vi "HFRR ADV v043.vi"() -> ()   [LabVIEW 2025] (continued)
                  n3190 = call-dynamic "Set Report Tab Width.vi"("report in"=w4006, "error in (no error)"=w4004) -> ("report out"=w4005:refnum<class "NI_report.lvclass">, "error out"=w4003:errorcluster)  [unwired: 12 in]
                }
                n3191 = local read "TITTLE"() -> (w3951:string)
                n3192 = call-dynamic "Set Report Header Text.vi"("report in"=w3934, "center header text"=w3951, "error in (no error)"=w3933) -> ("report out"=w3972:refnum<class "NI_report.lvclass">, "error out"=w3971:errorcluster)  [unwired: 11 in]
                n3193 = for {
                  N: 1 -> [_]
                  tunnel: [w4010] -> w3958
                  tunnel: [w4009] -> w3957
                  tunnel: w3972 -> [w4008]
                  tunnel: w3971 -> [w4007]
                  n3194 = call-dynamic "New Report Line.vi"("report in"=w4008, "error in (no error)"=w4007) -> ("report out"=w4010:refnum<class "NI_report.lvclass">, "error out"=w4009:errorcluster)  [unwired: 12 in]
                }
                n3195 = for {
                  N: 2 -> [_]
                  tunnel: [w4002] -> w3964
                  tunnel: [w4001] -> w3963
                  tunnel: w3958 -> [w4000]
                  tunnel: w3957 -> [w3999]
                  n3196 = call-dynamic "New Report Line.vi"("report in"=w4000, "error in (no error)"=w3999) -> ("report out"=w4002:refnum<class "NI_report.lvclass">, "error out"=w4001:errorcluster)  [unwired: 12 in]
                }
                n3197 = for {
                  N: 25 -> [_]
                  tunnel: w3964 -> [w3998]
                  tunnel: w3963 -> [w3996]
                  tunnel: [w3997] -> w3967
                  tunnel: [w3995] -> w3966
                  n3198 = call-dynamic "Set Report Tab Width.vi"("report in"=w3998, "error in (no error)"=w3996) -> ("report out"=w3997:refnum<class "NI_report.lvclass">, "error out"=w3995:errorcluster)  [unwired: 12 in]
                }
                n3199 = control-ref of="Tab Control 9"() -> (w3962:refnum<vi>)
                n3200 = call-dynamic "Append Control Image to Report.vi"("report in"=w3967, "alignment (default)"=HTML_Report_Image_Alignment."ABSMIDDLE", "ctrl reference"=w3962, "error in (no error)"=w3966) -> ("report out"=w3961:refnum<class "NI_report.lvclass">, "error out"=w3960:errorcluster)  [unwired: 8 in, 2 out]
                n3201 = for {
                  N: 3 -> [_]
                  tunnel: [w3994] -> w3945
                  tunnel: [w3993] -> w3944
                  tunnel: w3961 -> [w3992]
                  tunnel: w3960 -> [w3991]
                  n3202 = call-dynamic "New Report Line.vi"("report in"=w3992, "error in (no error)"=w3991) -> ("report out"=w3994:refnum<class "NI_report.lvclass">, "error out"=w3993:errorcluster)  [unwired: 12 in]
                }
                n3203 = for {
                  N: 100 -> [_]
                  tunnel: w3945 -> [w3990]
                  tunnel: w3944 -> [w3988]
                  tunnel: [w3989] -> w3941
                  tunnel: [w3987] -> w3939
                  n3204 = call-dynamic "Set Report Tab Width.vi"("report in"=w3990, "error in (no error)"=w3988) -> ("report out"=w3989:refnum<class "NI_report.lvclass">, "error out"=w3987:errorcluster)  [unwired: 12 in]
                }
                n3205 = String To Path(string="C:\\LAB-IQ\\im\\Temp_resized.jpg") -> (path=w3931:path)
                n3206 = call-poly <vilib>:"Append Image to Report.vi"("report in"=w3941, "path or URL of image"=w3931, "error in (no error)"=w3939) -> ("report out"=w3940:refnum<class "NI_report.lvclass">, "error out"=w3938:errorcluster)  [unwired: 9 in, 2 out]
                n3207 = call-poly <vilib>:"Open HTML Report in Browser.vi"("report in"=w3940, "error in (no error)"=w3938) -> ("report out"=w3975:refnum<class "NI_report.lvclass">, "error out"=w3974:errorcluster)  [unwired: 11 in, 1 out]
                n3208 = call-dynamic "Dispose Report.vi"("report in"=w3975, "error in (no error)"=w3974) -> ()  [unwired: 13 in, 1 out]
              }
              frame #2 {
              }
              frame #3 {
                n3209 = disable-structure shown="Disabled" {
                  frame Disabled {
                    n3210 = local read "String 10"() -> (w4015:string)
                    n3211 = Concatenate Strings("C:\\LAB-IQ-NXT\\Data\\" ("string"), w4015, ".jpg" ("string")) -> (w4013:string)
                    n3212 = String To Path(string=w4013) -> (path=w4012:path)
                    n3213 = Delete(path (use dialog)=w4012) -> ()  [unwired: 4 in, 3 out]
                  }
                  frame Enabled {
                  }
                }
                n3214 = local write "Print 2"(FALSE ("Print")) -> ()
              }
            }
          }
        }
      }
    }
    n3215 = Wait (ms)(milliseconds to wait=u32 50) -> ()  [unwired: 1 out]
    n3216 = Wait (ms)(milliseconds to wait=u32 50) -> ()  [unwired: 1 out]
    n3217 = local read "Quit"() -> (w2357:bool)
  }
  n3218 = VISA Close(VISA resource name=w45, error in (no error)=w44) -> ()  [unwired: 1 out]
  n3219 = while {
    stop <- w4166 stop-if-true
    n3220 = local read "Auto Start Test"() -> (w4164:bool)
    n3221 = local read "RUN"() -> (w4163:bool)
    n3222 = Wait (ms)(milliseconds to wait=u32 1000) -> ()  [unwired: 1 out]
    n3223 = Or(x=w4163, y=w4164) -> (x .or. y?=w4162:bool)
    n3224 = case shown="True" w4162 {
      frame False {
      }
      frame True {
        n3225 = local read "LVDT STROKE Actual"() -> (w4167:dbl)
        n3226 = In Range and Coerce(upper limit=1.2, x=w4167, lower limit=0.6) -> (In Range?=w4170:bool)  [unwired: 1 out]
        n3227 = call-poly <vilib>:"Random Number (Range).vi"("lower bound (0)"=0.998 ("upper bound (100)"), "upper bound (100)"=1.003) -> ("number"=w4168:dbl)  [unwired: 9 in]
        n3228 = case shown="True" w4170 {
          tunnel: [w4175 w4176] -> w4169
          tunnel: w4168 -> [_ w4176]
          tunnel: w4167 -> [w4175 _]
          frame False {
          }
          frame True {
          }
        }
        "LVDT STROKE DISPLAY" <- w4169
      }
    }
    n3229 = local read "Quit"() -> (w4166:bool)
  }
  n3230 = while {
    tunnel: [w4193] -> w53
    shift-right: [w4186] -> _
    shift-left: 0.0 -> [w4189]
    shift-right: [w4185] -> _
    shift-left: 0.0 -> [w4188]
    shift-right: [w4184] -> _
    shift-left: 100.0 ("vc_cmd") -> [w4187]
    stop <- w4193 stop-if-true
    # "PID LOGIC"
    n3231 = local read "run test Calibration"() -> (w4181:bool)
    n3232 = local read "RUN"() -> (w4191:bool)
    n3233 = local read "Auto Start Temp"() -> (w4182:bool)
    n3234 = local read "Auto Start Test"() -> (w4190:bool)
    n3235 = local read "START TEMP"() -> (w4180:bool)
    n3236 = And(x=w4182, y=w4190) -> (x .and. y?=w4183:bool)
    n3237 = Or(x=w4191, y=w4183) -> (x .or. y?=w4192:bool)
    n3238 = And(x=w4192, y=w4180) -> (x .and. y?=w4179:bool)
    n3239 = And(x=w4181, y=w4180) -> (x .and. y?=w4178:bool)
    n3240 = Or(x=w4178, y=w4179) -> (x .or. y?=w4177:bool)
    n3241 = Wait (ms)(milliseconds to wait="milliseconds to wait") -> ()  [unwired: 1 out]
    n3242 = case shown="True" w4177 {
      tunnel: [400.0 ("out_vc_cmd") w4212] -> w4184
      tunnel: [w4196 w4214] -> w4185
      tunnel: [w4196 w4213] -> w4186
      tunnel: w4189 -> [_ w4203]
      tunnel: w4188 -> [_ w4202]
      tunnel: w4187 -> [_ w4201]
      tunnel: w4181 -> [_ w4197]
      frame False {
        w4196 = 0.0 ("error_out")
      }
      frame True {
        n3243 = case shown="True" w4197 {
          tunnel: [w4221 1.0] -> w4199
          frame False {
            n3244 = local read "Set Strk"() -> (w4220:dbl)
            n3245 = Add(x=w4220, y="Add up Stroke") -> (x+y=w4221:dbl)
          }
          frame True {
          }
        }
        n3246 = local read "LVDT STROKE"() -> (w4198:dbl)
        n3247 = formula code="// Zero-Hardcode Explicit Positional-Form PID Engine\n// Inputs: target_stroke, measured_stroke, dt, prev_error, integral_accumulator_in, prev_vc_cmd\n//         kp, ki, kd, max_step_change, max_amplitude, min_amplitude, startup_cmd\n// Outputs: vc_cmd, error_out, out_error, integral_accumulator_out, out_vc_cmd\n\n// 1. Calculate Tracking Error\nfloat current_error = target_stroke - measured_stroke;\nerror_out = current_error;\n\n// 2. Compute Proportional Term\nfloat p_term = kp * current_error;\n\n// 3. Compute Derivative Term\nfloat d_term = 0.0;\nif (dt > 0.0) {\n    d_term = kd * ((current_error - prev_error) / dt);\n}\n\n// 4. Update and Accumulate Integral Term\nfloat current_integral = integral_accumulator_in + (current_error * dt);\nfloat i_term = ki * current_integral;\n\n// 5. Calculate Ideal Target Command (Anchored by startup baseline)\nfloat ideal_command = startup_cmd + p_term + i_term + d_term;\n\n// 6. Apply Loop Rate Limiting FIRST \n// (Forces the command to climb gradually from prev_vc_cmd instead of jumping straight to max)\nfloat raw_adjustment = ideal_command - prev_vc_cmd;\n\nif (raw_adjustment > max_step_change) {\n    raw_adjustment = max_step_change;\n} else if (raw_adjustment < -max_step_change) {\n    raw_adjustment = -max_step_change;\n}\n\nfloat next_vc_cmd = prev_vc_cmd + raw_adjustment;\n\n// 7. Anti-Windup Protection & Final Output Safety Safeguard Clamping\n// (Back-calculating based on what we are ACTUALLY outputting)\nif (next_vc_cmd > max_amplitude) {\n    float excess = next_vc_cmd - max_amplitude;\n    if (ki > 0.0) {\n        current_integral -= excess / ki;\n    }\n    next_vc_cmd = max_amplitude;\n} else if (next_vc_cmd < min_amplitude) {\n    float excess = next_vc_cmd - min_amplitude;\n    if (ki > 0.0) {\n        current_integral -= excess / ki;\n    }\n    next_vc_cmd = min_amplitude;\n}\n\n// 8. Map to Shift Registers for memory persistence\nvc_cmd = next_vc_cmd;\nout_error = current_error;                   \nintegral_accumulator_out = current_integral;  \nout_vc_cmd = next_vc_cmd;"("target_stroke"=w4199, "measured_stroke"=w4198, "dt"="dt", "integral_accumulator_in"=w4202, "prev_error"=w4203, "prev_vc_cmd"=w4201, "kp"="kp", "ki"="ki", "kd"="kd", "max_step_change"="max_step_change", "max_amplitude"="max_amplitude", "min_amplitude"="min_amplitude", "startup_cmd"="startup_cmd") -> ("vc_cmd"=w4218:dbl, "out_error"=w4213:dbl, "integral_accumulator_out"=w4214:dbl, "out_vc_cmd"=w4212:dbl)  [unwired: 1 out]
        "output Vpp" <- w4218
        n3248 = Number To Fractional String(number=w4218, precision (6)=i16 1) -> (F-format string=w4216:string)  [unwired: 2 in]
        n3249 = Concatenate Strings("DAC;" ("string"), w4216) -> (w4200:string)
        n3250 = local write "Due Write"(w4200) -> ()
        "prev_error" <- w4203
        "integral_accumulator_in" <- w4202
        "prev_vc_cmd" <- w4201
      }
    }
    n3251 = local read "Quit"() -> (w4193:bool)
  }
  n3252 = Or(x=w49, y=w48) -> (x .or. y?=w50:bool)
  n3253 = Or(x=w46, y=w50) -> (x .or. y?=w55:bool)
  n3254 = control-ref of="new picture"() -> ()  [unwired: 1 out]
  n3255 = Or(x=w58, y=w55) -> (x .or. y?=w52:bool)
  n3256 = Or(x=w52, y=w53) -> (x .or. y?=w47:bool)
  n3257 = while {
    tunnel: [w4223] -> w57
    i -> [w4230]
    stop <- w4223 stop-if-true
    n3258 = local read "Quit"() -> (w4223:bool)
    n3259 = Equal To 0?(x=w4230) -> (x = 0?=w4228:bool)
    n3260 = call "Elapsed Time3"("Time Target (s)"=45.0, "Auto Reset"=TRUE) -> ("Time has Elapsed"=w4227:bool)  [unwired: 10 in, 7 out]
    n3261 = Wait (ms)(milliseconds to wait=u32 50) -> ()  [unwired: 1 out]
    n3262 = Or(x=w4227, y=w4228) -> (x .or. y?=w4229:bool)
    n3263 = case shown="True" w4229 {
      frame False {
      }
      frame True {
        n3264 = call <vilib>:"System Exec.vi"("run minimized? (F)"=TRUE, "error in (no error)"="error in (no error)", "command line"="powercfg.exe -change -monitor-timeout-ac 0") -> ("error out"=w4241:errorcluster)  [unwired: 5 in, 3 out]
        n3265 = call <vilib>:"System Exec.vi"("run minimized? (F)"=TRUE, "error in (no error)"=w4241, "command line"="powercfg.exe -change -disk-timeout-ac 0") -> ("error out"=w4240:errorcluster)  [unwired: 5 in, 3 out]
        n3266 = call <vilib>:"System Exec.vi"("run minimized? (F)"=TRUE, "error in (no error)"=w4240, "command line"="powercfg.exe -change -standby-timeout-ac 0") -> ("error out"=w4239:errorcluster)  [unwired: 5 in, 3 out]
        n3267 = call <vilib>:"System Exec.vi"("run minimized? (F)"=TRUE, "error in (no error)"=w4239, "command line"="powercfg.exe -change -hibernate-timeout-ac 0") -> ("error out"=w4238:errorcluster)  [unwired: 5 in, 3 out]
        n3268 = call <vilib>:"Simple Error Handler.vi"("error in (no error)"=w4238) -> ("error out"=w4244:errorcluster)  [unwired: 4 in, 4 out]
        n3269 = call <vilib>:"Clear Errors.vi"("error in (no error)"=w4244) -> ("error out"=→"error out":errorcluster)  [unwired: 5 in, 1 out]
      }
    }
  }
  n3270 = Compound Arithmetic op=OR(w60, w47, w57) -> (w59:bool)
  n3271 = flat-sequence {
    tunnel: w59 -> [_]
    tunnel: [w4246] -> w29
    tunnel: w29 -> [_]
    frame #0 {
      n3272 = call "CLOSE CONNECTION.vi"() -> ("error out"=w4246:errorcluster)  [unwired: 11 in]
    }
    frame #1 {
      n3273 = Quit LabVIEW(quit? (T)=TRUE) -> ()
      n3274 = local write "Quit"(FALSE ("EXIT")) -> ()
    }
  }
  n3275 = property on="Heater Button" class="Bool (strict)"("Visible"=TRUE) -> ()  [unwired: 2 in, 2 out]
  n3276 = while {
    tunnel: [w4253] -> _
    i -> [w4253]
    stop <- w4249 stop-if-true
    # "Langauage selection"
    n3277 = Equal?(x="Lan flag", y=22.0) -> ()  [unwired: 1 out]
    n3278 = disable-structure shown="Disabled" {
      frame Disabled {
        n3279 = stacked-sequence {
          frame #0 {
            n3280 = case shown="\"Russian\"" "Language Selection" {
              tunnel: [0 1] -> w4255
              frame "English", Default {
              }
              frame "Russian" {
              }
            }
            n3281 = for {
              N: 130 -> [_]
              tunnel: "Table" -> [w4264]
              tunnel: w4255 -> [w4263]
              i -> [w4262]
              n3282 = Index Array(array=w4264, index (row)=w4262, index (col)=w4263) -> (element=w4261:string)
              n3283 = case shown="1" w4262 {
                tunnel: w4261 -> [w4265 w4266 _ w4267 w4268 w4269 w4270 w4271 w4272 w4273 w4274 w4275 w4276 w4277 w4278 w4279 w4280 w4281 w4282 w4283 w4284 w4285 w4286 w4287 w4288 w4289 w4290 w4291 w4292 _ _ w4293 w4294 w4295 w4296 w4297 w4298 w4307 w4314 w4321 w4328 w4332 w4335 w4338 w4340 w4342 w4343 w4344 w4345 w4346 w4347 w4348 w4349 w4350 w4351 w4352 w4353 w4354 w4355 w4356 w4357 w4358 w4359 w4360 w4361 w4362 w4363 w4364 w4365 w4366 w4367 w4368 w4369 w4370 w4371 w4372 w4373 w4374 w4375 w4376 w4377 w4378 w4379 w4380 w4381 w4382 w4383 w4384 w4385 w4386 w4387 w4388 w4389 w4390 w4391 w4392 w4393 w4394 w4395 w4396 w4397 w4398 w4399 w4400 w4401 _ w4402 w4403 w4404 w4405 w4406 w4407 w4408 w4409 w4410 w4411 w4412 w4413 w4414 _ w4415 w4416 w4417 w4418 w4419 w4420 _]
                frame 0 {
                  n3284 = local write "S"(w4265) -> ()
                }
                frame 1 {
                  n3285 = local write "S 2"(w4266) -> ()
                }
                frame 2 {
                }
                frame 3 {
                  n3286 = local write "S 4"(w4267) -> ()
                }
                frame 4 {
                  n3287 = property on="FILE" class="Str"("Caption.Text"=w4268) -> ()  [unwired: 2 in, 2 out]
                }
                frame 5 {
                  n3288 = property on="Fuel Discription :" class="Str"("Caption.Text"=w4269) -> ()  [unwired: 2 in, 2 out]
                }
                frame 6 {
                  n3289 = property on="Remarks :" class="Str"("Caption.Text"=w4270) -> ()  [unwired: 2 in, 2 out]
                }
                frame 7 {
                  n3290 = property on="Save & Continue" class="Bool (strict)"("Boolean Text.Text"=w4271) -> ()  [unwired: 2 in, 2 out]
                }
                frame 8 {
                }
                frame 9 {
                  n3291 = property on="Set Hz" class="DigNum (strict)"("Caption.Text"=w4273) -> ()  [unwired: 2 in, 2 out]
                }
                frame 10 {
                }
                frame 11 {
                  n3292 = property on="NORMAL LOAD" class="DigNum (strict)"("Caption.Text"=w4275) -> ()  [unwired: 2 in, 2 out]
                }
                frame 12 {
                }
                frame 13 {
                  n3293 = property on="Set Temp" class="DigNum (strict)"("Caption.Text"=w4277) -> ()  [unwired: 2 in, 2 out]
                }
                frame 14 {
                  n3294 = local write "S 15"(w4278) -> ()
                }
                frame 15 {
                  n3295 = property on="Set Rh" class="DigNum (strict)"("Caption.Text"=w4279) -> ()  [unwired: 2 in, 2 out]
                }
                frame 16 {
                }
                frame 17 {
                  n3296 = local write "S 18"(w4281) -> ()
                }
                frame 18 {
                  "String 17" <- w4282
                }
                frame 19 {
                  n3297 = property on="test time" class="DigNum (strict)"("Caption.Text"=w4283) -> ()  [unwired: 2 in, 2 out]
                }
                frame 20 {
                  "String 18" <- w4284
                  "String 22" <- w4284
                }
                frame 21 {
                  n3298 = property on="Elapsed time" class="DigNum (strict)"("Caption.Text"=w4285) -> ()  [unwired: 2 in, 2 out]
                }
                frame 22 {
                  n3299 = property on="Samplingtime 2" class="DigNum (strict)"("Caption.Text"=w4286) -> ()  [unwired: 2 in, 2 out]
                }
                frame 23 {
                  "String 21" <- w4287
                }
                frame 24 {
                  n3300 = property on="Countdown" class="DigNum (strict)"("Caption.Text"=w4288) -> ()  [unwired: 2 in, 2 out]
                }
                frame 25 {
                  n3301 = property on="Countdown 2" class="DigNum (strict)"("Caption.Text"=w4289) -> ()  [unwired: 2 in, 2 out]
                }
                frame 26 {
                  n3302 = property on="Engage" class="Bool (strict)"("Boolean Text.Text"=w4290) -> ()  [unwired: 2 in, 2 out]
                }
                frame 27 {
                  n3303 = property on="Boolean  4" class="Bool (strict)"("Boolean Text.Text"=w4291) -> ()  [unwired: 2 in, 2 out]
                }
                frame 28 {
                  n3304 = property on="Test \nStatus" class="Bool (strict)"("Boolean Text.Text"=w4292) -> ()  [unwired: 2 in, 2 out]
                }
                frame 29 {
                }
                frame 30 {
                }
                frame 31 {
                }
                frame 32 {
                  n3305 = property on="RSTCOF" class="Bool"("Boolean Text.Text"=w4294) -> ()  [unwired: 2 in, 2 out]
                  n3306 = property on="RST FF" class="Bool"("Boolean Text.Text"=w4294) -> ()  [unwired: 2 in, 2 out]
                  n3307 = property on="RST TEMP" class="Bool"("Boolean Text.Text"=w4294) -> ()  [unwired: 2 in, 2 out]
                  n3308 = property on="RSTV1 3" class="Bool"("Boolean Text.Text"=w4294) -> ()  [unwired: 2 in, 2 out]
                  n3309 = property on="rstv2" class="Bool"("Boolean Text.Text"=w4294) -> ()  [unwired: 2 in, 2 out]
                  n3310 = property on="RSTV1 2" class="Bool"("Boolean Text.Text"=w4294) -> ()  [unwired: 2 in, 2 out]
                  n3311 = property on="RST CP" class="Bool"("Boolean Text.Text"=w4294) -> ()  [unwired: 2 in, 2 out]
                }
                frame 33 {
                  "S 61" <- w4295
                }
                frame 34 {
                  "String 23" <- w4296
                }
                frame 35 {
                  n3312 = property on="Rh Before" class="DigNum (strict)"("Caption.Text"=w4297) -> ()  [unwired: 2 in, 2 out]
                }
                frame 36 {
                  n3313 = Match Pattern(string=w4298, regular expression=",") -> (before substring=→"bs":string, after substring=→"as":string)  [unwired: 1 in, 2 out]
                  n3314 = property on="Rh After" class="DigNum (strict)"("Caption.Text"=w4298) -> ()  [unwired: 2 in, 2 out]
                }
                frame 37 {
                  n3315 = Match Pattern(string=w4307, regular expression=",") -> (before substring=w4306:string, after substring=w4305:string)  [unwired: 1 in, 2 out]
                  "bs" <- w4306
                  "as" <- w4305
                  n3316 = Concatenate Strings(w4306, w4305) -> (w4302:string)
                  n3317 = property on="Humidity before test 2" class="DigNum (strict)"("Caption.Text"=w4302) -> ()  [unwired: 2 in, 2 out]
                  n3318 = Concatenate Strings(w4302, "=" ("string")) -> (w4303:string)
                  n3319 = local write "S 38"(w4303) -> ()
                }
                frame 38 {
                  n3320 = Match Pattern(string=w4314, regular expression=",") -> (before substring=w4313:string, after substring=w4312:string)  [unwired: 1 in, 2 out]
                  "bs" <- w4313
                  "as" <- w4312
                  n3321 = Concatenate Strings(w4313, w4312) -> (w4309:string)
                  n3322 = property on="Humidity after test 2" class="DigNum (strict)"("Caption.Text"=w4309) -> ()  [unwired: 2 in, 2 out]
                  n3323 = Concatenate Strings(w4309, "=" ("string")) -> (w4311:string)
                  n3324 = local write "S 39"(w4311) -> ()
                }
                frame 39 {
                  n3325 = Match Pattern(string=w4321, regular expression=",") -> (before substring=w4320:string, after substring=w4319:string)  [unwired: 1 in, 2 out]
                  "bs" <- w4320
                  "as" <- w4319
                  n3326 = Concatenate Strings(w4320, w4319) -> (w4316:string)
                  n3327 = property on="Temperature before test 2" class="DigNum (strict)"("Caption.Text"=w4316) -> ()  [unwired: 2 in, 2 out]
                  n3328 = Concatenate Strings(w4316, "=" ("string")) -> (→"String 34":string)
                }
                frame 40 {
                  n3329 = Match Pattern(string=w4328, regular expression=",") -> (before substring=w4327:string, after substring=w4326:string)  [unwired: 1 in, 2 out]
                  "bs" <- w4327
                  "as" <- w4326
                  n3330 = Concatenate Strings(w4327, w4326) -> (w4323:string)
                  n3331 = property on="Temperature after test 2" class="DigNum (strict)"("Caption.Text"=w4323) -> ()  [unwired: 2 in, 2 out]
                  n3332 = Concatenate Strings(w4323, "=" ("string")) -> (→"String 35":string)
                  n3333 = property on="Temperature after test" class="DigNum (strict)"("Caption.Text"=w4323) -> ()  [unwired: 2 in, 2 out]
                }
                frame 41 {
                  n3334 = property on="AVP 2" class="DigNum (strict)"("Caption.Text"=w4332) -> ()  [unwired: 2 in, 2 out]
                  n3335 = Concatenate Strings(w4332, "=" ("string")) -> (→"String 36":string)
                }
                frame 42 {
                  n3336 = property on="MWSD 2" class="DigNum (strict)"("Caption.Text"=w4335) -> ()  [unwired: 2 in, 2 out]
                  n3337 = Concatenate Strings(w4335, "=" ("string")) -> (→"String 37":string)
                }
                frame 43 {
                  n3338 = property on="HCF 2" class="DigNum (strict)"("Caption.Text"=w4338) -> ()  [unwired: 2 in, 2 out]
                  n3339 = Concatenate Strings(w4338, "=" ("string")) -> (→"String 38":string)
                }
                frame 44 {
                  n3340 = Concatenate Strings(w4340, "=" ("string")) -> (→"String 39":string)
                  n3341 = property on="WS1.4 2" class="DigNum (strict)"("Caption.Text"=w4340) -> ()  [unwired: 2 in, 2 out]
                }
                frame 45 {
                }
                frame 46 {
                  n3342 = local write "S 47"(w4343) -> ()
                }
                frame 47 {
                  n3343 = local write "S 48"(w4344) -> ()
                }
                frame 48 {
                  n3344 = local write "S 49"(w4345) -> ()
                }
                frame 49 {
                  n3345 = local write "S 50"(w4346) -> ()
                }
                frame 50 {
                  n3346 = local write "S 51"(w4347) -> ()
                }
                frame 51 {
                  n3347 = local write "S 52"(w4348) -> ()
                }
                frame 52 {
                  n3348 = local write "S 53"(w4349) -> ()
                }
                frame 53 {
                  n3349 = local write "S 54"(w4350) -> ()
                }
                frame 54 {
                  n3350 = local write "S 55"(w4351) -> ()
                }
                frame 55 {
                  n3351 = local write "S 56"(w4352) -> ()
                }
                frame 56 {
                  n3352 = local write "S 57"(w4353) -> ()
                }
                frame 57 {
                  n3353 = local write "S 58"(w4354) -> ()
                }
                frame 58 {
                  n3354 = local write "S 59"(w4355) -> ()
                }
                frame 59 {
                  n3355 = local write "S 60"(w4356) -> ()
                }
                frame 60 {
                  n3356 = local write "S 62"(w4357) -> ()
                }
                frame 61 {
                  n3357 = local write "S 63"(w4358) -> ()
                }
                frame 62 {
                  n3358 = local write "S 64"(w4359) -> ()
                }
                frame 63 {
                  n3359 = local write "S 65"(w4360) -> ()
                }
                frame 64 {
                  n3360 = local write "S 66"(w4361) -> ()
                }
                frame 65 {
                  n3361 = local write "S 67"(w4362) -> ()
                }
                frame 66 {
                  n3362 = local write "S 68"(w4363) -> ()
                }
                frame 67 {
                  n3363 = local write "S 69"(w4364) -> ()
                }
                frame 68 {
                  n3364 = local write "S 70"(w4365) -> ()
                }
                frame 69 {
                  n3365 = local write "S 71"(w4366) -> ()
                }
                frame 70 {
                  n3366 = local write "S 72"(w4367) -> ()
                }
                frame 71 {
                  n3367 = local write "S 73"(w4368) -> ()
                }
                frame 72 {
                  n3368 = local write "S 74"(w4369) -> ()
                }
                frame 73 {
                  n3369 = local write "S 75"(w4370) -> ()
                }
                frame 74 {
                  n3370 = local write "S 76"(w4371) -> ()
                }
                frame 75 {
                  n3371 = local write "S 77"(w4372) -> ()
                }
                frame 76 {
                  n3372 = local write "S 78"(w4373) -> ()
                }
                frame 77 {
                  n3373 = local write "S 79"(w4374) -> ()
                }
                frame 79 {
                  n3374 = property on="Sample Temperature ( °C )" class="XYGraph (strict)"("Y Scale.Name Label.Text"=w4375) -> ()  [unwired: 2 in, 2 out]
                }
                frame 80 {
                  n3375 = local write "S 81"(w4376) -> ()
                  n3376 = property on="Humidity ( %RH )" class="XYGraph (strict)"("Y Scale.Name Label.Text"=w4376) -> ()  [unwired: 2 in, 2 out]
                }
                frame 78 {
                  n3377 = property on="Air Temperature  ( °C )" class="XYGraph (strict)"("X Scale.Name Label.Text"=w4377) -> ()  [unwired: 2 in, 2 out]
                  n3378 = property on="Humidity ( %RH )" class="XYGraph (strict)"("X Scale.Name Label.Text"=w4377) -> ()  [unwired: 2 in, 2 out]
                  n3379 = property on="Sample Temperature ( °C )" class="XYGraph (strict)"("X Scale.Name Label.Text"=w4377) -> ()  [unwired: 2 in, 2 out]
                  n3380 = property on="Coefficient Of Friction" class="XYGraph (strict)"("X Scale.Name Label.Text"=w4377) -> ()  [unwired: 2 in, 2 out]
                }
                frame 81 {
                  n3381 = property on="Air Temperature  ( °C )" class="XYGraph (strict)"("Y Scale.Name Label.Text"=w4378) -> ()  [unwired: 2 in, 2 out]
                }
                frame 82 {
                  n3382 = local write "S 84"(w4379) -> ()
                }
                frame 83 {
                  n3383 = local write "S 85"(w4380) -> ()
                }
                frame 84 {
                  n3384 = local write "S 86"(w4381) -> ()
                }
                frame 85 {
                  n3385 = local write "S 87"(w4382) -> ()
                }
                frame 86 {
                  n3386 = local write "S 88"(w4383) -> ()
                }
                frame 87 {
                }
                frame 88 {
                  n3387 = local write "S 90"(w4385) -> ()
                }
                frame 89 {
                  n3388 = local write "S 91"(w4386) -> ()
                }
                frame 90 {
                  n3389 = local write "S 92"(w4387) -> ()
                }
                frame 91 {
                  n3390 = local write "S 93"(w4388) -> ()
                }
                frame 92 {
                  n3391 = local write "S 94"(w4389) -> ()
                }
                frame 93 {
                  n3392 = local write "S 95"(w4390) -> ()
                }
                frame 94 {
                  n3393 = local write "S 96"(w4391) -> ()
                }
                frame 95 {
                  n3394 = local write "S 97"(w4392) -> ()
                }
                frame 96 {
                  n3395 = local write "S 98"(w4393) -> ()
                }
                frame 97 {
                  n3396 = local write "S 99"(w4394) -> ()
                }
                frame 98 {
                  n3397 = local write "S 100"(w4395) -> ()
                }
                frame 99 {
                  n3398 = local write "S 101"(w4396) -> ()
                }
                frame 100 {
                  n3399 = local write "S 102"(w4397) -> ()
                }
                frame 101 {
                  n3400 = local write "S 103"(w4398) -> ()
                }
                frame 102 {
                  n3401 = local write "S 104"(w4399) -> ()
                }
                frame 103 {
                  n3402 = local write "S 105"(w4400) -> ()
                }
                frame 104 {
                  n3403 = local write "S 106"(w4401) -> ()
                }
                frame 105 {
                }
                frame 106 {
                  n3404 = property on="OK Button 17" class="Bool (strict)"("Boolean Text.Text"=w4402) -> ()  [unwired: 2 in, 2 out]
                }
                frame 107 {
                  n3405 = property on="OK Button 16" class="Bool (strict)"("Boolean Text.Text"=w4403) -> ()  [unwired: 2 in, 2 out]
                }
                frame 108 {
                  n3406 = property on="TITTLE" class="Str"("Caption.Text"=w4404) -> ()  [unwired: 2 in, 2 out]
                }
                frame 109 {
                  "String 30" <- w4405
                }
                frame 110 {
                  n3407 = property on="Test Date" class="Str"("Caption.Text"=w4406) -> ()  [unwired: 2 in, 2 out]
                  "String 31" <- w4406
                }
                frame 111 {
                  n3408 = property on="Sample ID" class="Str"("Caption.Text"=w4407) -> ()  [unwired: 2 in, 2 out]
                  "String 32" <- w4407
                }
                frame 112 {
                  n3409 = property on="Tested by" class="Str"("Caption.Text"=w4408) -> ()  [unwired: 2 in, 2 out]
                  "String 33" <- w4408
                }
                frame 113 {
                  n3410 = property on="System Configured Printers 2" class="Arr (strict)"("Caption.Text"=w4409) -> ()  [unwired: 2 in, 2 out]
                }
                frame 114 {
                  n3411 = property on="Selected Printer" class="Str"("Caption.Text"=w4410) -> ()  [unwired: 2 in, 2 out]
                }
                frame 115 {
                  n3412 = property on="Select Printer 3" class="DigNum (strict)"("Caption.Text"=w4411) -> ()  [unwired: 2 in, 2 out]
                }
                frame 116 {
                  n3413 = property on="Print" class="Bool (strict)"("Boolean Text.Text"=w4412) -> ()  [unwired: 2 in, 2 out]
                }
                frame 117 {
                  "String 41" <- w4413
                }
                frame 118 {
                  n3414 = property on="tested by" class="Str"("Caption.Text"=w4414) -> ()  [unwired: 2 in, 2 out]
                }
                frame 119 {
                }
                frame 120 {
                  n3415 = property on="Export" class="Bool (strict)"("Boolean Text.Text"=w4415) -> ()  [unwired: 2 in, 2 out]
                }
                frame 121 {
                }
                frame 122 {
                }
                frame 123 {
                  n3416 = property on="Select File Type" class="Enum (strict)"("Caption.Text"=w4418) -> ()  [unwired: 2 in, 2 out]
                }
                frame 124 {
                  n3417 = property on="s.NO" class="Str"("Caption.Text"=w4419) -> ()  [unwired: 2 in, 2 out]
                  "String 45" <- w4419
                }
                frame 125 {
                  n3418 = property on="trip1 8" class="Bool (strict)"("Boolean Text.Text"=w4420) -> ()  [unwired: 2 in, 2 out]
                }
                frame 126, Default {
                }
              }
            }
          }
          frame #1 {
            w4428 = TRUE ("Visible")
            n3419 = local read "S 91"() -> (w4445:string)
            n3420 = local read "S 90"() -> (w4444:string)
            n3421 = local read "S 88"() -> (w4443:string)
            n3422 = property on="File Path" class="Path"("Caption.Text"=w4444) -> ()  [unwired: 2 in, 2 out]
            n3423 = local read "S 71"() -> (w4438:string)
            n3424 = local read "S 86"() -> (w4440:string)
            n3425 = local read "S 85"() -> (w4441:string)
            n3426 = local read "S 87"() -> (w4439:string)
            n3427 = local read "S 84"() -> (w4442:string)
            n3428 = local read "S 103"() -> (w4427:string)
            n3429 = local read "S 104"() -> (w4426:string)
            n3430 = property on="Password" class="Str"("Caption.Text"=w4441) -> ()  [unwired: 2 in, 2 out]
            n3431 = property on="EDIT" class="Bool (strict)"("Boolean Text.Text"=w4438) -> ()  [unwired: 2 in, 2 out]
            n3432 = property on="SAVE" class="Bool (strict)"("Boolean Text.Text"=w4442) -> ()  [unwired: 2 in, 2 out]
            n3433 = Build Array(w4427, w4426) -> (w4425:string[])
            n3434 = property on="Heater Button" class="Bool (strict)"("Strings [4]"=w4425) -> ()  [unwired: 2 in, 2 out]
            n3435 = local read "S 92"() -> (w4437:string)
            n3436 = local read "S 93"() -> (w4436:string)
            n3437 = local read "S 105"() -> (w4423:string)
            n3438 = local read "S 106"() -> (w4422:string)
            n3439 = Build Array(w4437, w4436) -> ()  [unwired: 1 out]
            n3440 = Build Array(w4423, w4422) -> (w4424:string[])
            n3441 = local read "S 95"() -> (w4434:string)
            n3442 = local read "S 94"() -> (w4435:string)
            n3443 = local read "bs"() -> (w4450:string)
            n3444 = local read "as"() -> (w4451:string)
            n3445 = property on="Humidity" class="Bool (strict)"("Strings [4]"=w4424) -> ()  [unwired: 2 in, 2 out]
            n3446 = Concatenate Strings(w4450, "\r", w4451) -> ()  [unwired: 1 out]
            n3447 = property on="Rh After" class="DigNum (strict)"("Caption.Size to Text?"=TRUE ("Caption.Size to Text")) -> ()  [unwired: 2 in, 2 out]
            n3448 = local read "S 48"() -> (w4474:string)
            n3449 = local read "S 50"() -> (w4472:string)
            n3450 = local read "S 51"() -> (w4471:string)
            n3451 = local read "S 49"() -> (w4473:string)
            n3452 = local read "S 52"() -> (w4470:string)
            n3453 = local read "as"() -> (w4455:string)
            n3454 = local read "bs"() -> (w4456:string)
            n3455 = local read "S 56"() -> (w4469:string)
            n3456 = local read "S 57"() -> (w4468:string)
            n3457 = local read "S 58"() -> (w4467:string)
            n3458 = local read "S 59"() -> (w4466:string)
            n3459 = property on="OPEN" class="Bool (strict)"("Boolean Text.Text"=w4470) -> ()  [unwired: 2 in, 2 out]
            n3460 = property on="OPEN 1" class="Bool (strict)"("Boolean Text.Text"=w4474) -> ()  [unwired: 2 in, 2 out]
            n3461 = property on="OPEN 2" class="Bool (strict)"("Boolean Text.Text"=w4473) -> ()  [unwired: 2 in, 2 out]
            n3462 = property on="OPEN 3" class="Bool (strict)"("Boolean Text.Text"=w4472) -> ()  [unwired: 2 in, 2 out]
            n3463 = property on="OPEN 4" class="Bool (strict)"("Boolean Text.Text"=w4471) -> ()  [unwired: 2 in, 2 out]
            n3464 = Concatenate Strings(w4456, "\r", w4455) -> ()  [unwired: 1 out]
            n3465 = local read "S 102"() -> (w4429:string)
            n3466 = property on="КОФ1" class="DigNum (strict)"("Caption.Text"=w4469) -> ()  [unwired: 2 in, 2 out]
            n3467 = local read "S 98"() -> (w4433:string)
            n3468 = local read "S 99"() -> (w4432:string)
            n3469 = local read "S 100"() -> (w4431:string)
            n3470 = local read "S 101"() -> (w4430:string)
            n3471 = property on="КОФ2" class="DigNum (strict)"("Caption.Text"=w4468) -> ()  [unwired: 2 in, 2 out]
            n3472 = property on="КОФ3" class="DigNum (strict)"("Caption.Text"=w4467) -> ()  [unwired: 2 in, 2 out]
            n3473 = property on="КОФ4" class="DigNum (strict)"("Caption.Text"=w4466) -> ()  [unwired: 2 in, 2 out]
            n3474 = local read "bs"() -> (w4454:string)
            n3475 = local read "as"() -> (w4453:string)
            n3476 = local read "S 60"() -> (w4465:string)
            n3477 = local read "S 54"() -> (w4475:string)
            n3478 = Concatenate Strings(w4454, "\r", w4453) -> ()  [unwired: 1 out]
            n3479 = Concatenate Strings(w4475, w4465) -> ()  [unwired: 1 out]
            n3480 = local read "S 77"() -> (→"String 43":string)
            n3481 = local read "S 76"() -> (w4448:string)
            n3482 = local read "S 78"() -> (w4447:string)
            n3483 = local read "S 71"() -> (w4459:string)
            n3484 = local read "S 66"() -> (w4464:string)
            n3485 = local read "S 67"() -> (w4463:string)
            n3486 = local read "S 68"() -> (w4462:string)
            n3487 = local read "S 69"() -> (w4461:string)
            n3488 = local read "S 70"() -> (w4460:string)
            n3489 = property on="AIR TEMP" class="DigNum (strict)"("Caption.Text"=w4447) -> ()  [unwired: 2 in, 2 out]
            n3490 = property on="Set Strk" class="DigNum (strict)"("Caption.Text"=w4448) -> ()  [unwired: 2 in, 2 out]
            n3491 = property on="SPEED OUT:" class="DigNum (strict)"("Caption.Text"=w4462) -> ()  [unwired: 2 in, 2 out]
            n3492 = property on="EDIT" class="Bool (strict)"("Boolean Text.Text"=w4459) -> ()  [unwired: 2 in, 2 out]
            n3493 = local read "S 79"() -> (w4446:string)
          }
          frame #2 {
          }
        }
        n3494 = local write "Lan flag"(10.0 ("Lan flag")) -> ()
      }
      frame Enabled {
      }
    }
    n3495 = Wait (ms)(milliseconds to wait=u32 2000) -> ()  [unwired: 1 out]
    n3496 = local read "Quit"() -> (w4249:bool)
  }
  n3497 = while {
    shift-right: [w4481] -> _
    shift-left: _ -> [w4482]
    shift-right: [w4479] -> _
    shift-left: T18 {"Read Heave and Surge"="", "Bytes at Heave Port"=0.0, "Heave and Surge COM Port:"="COM9", "Com Port 2"="COM7", "Residual Due"="", "Heave COM Status 2"=TRUE, "Heave COM Status"=TRUE, "Port 2"=TRUE, "Sway PPR"=6400.0, "Surge PPR"=6400.0, "Heave PPR"=6400.0, "Sway Pitch"=2.0, "Surge Pitch"=3.0, "Heave Pitch"=4.0, "Sway Pulses/mm"=320.0, "Surge Pulses/mm"=1600.0, "Heave Pulses/mm"=1600.0, "inner loop"=0.0, "Read Heave and Surge 2"="", "String 36"="", "Write S"=FALSE, "WriteCC1"=[""], "Heave COM Loop"=0, "LastCom"="", "EXIT"=FALSE, "Error Heave"={"status"=TRUE, "code"=-1073807343, "source"=""}} -> [w4478]
    shift-right: [w4476] -> _
    shift-left: enum16{"init", "MAIN", "Panel Close"}."init" -> [w4477]
    stop <- w4480 stop-if-true
    # "HUMIDITY LOOP LOGIC"
    n3498 = case shown="\"MAIN\"" w4477 {
      tunnel: w4482 -> [w4496 w4520 w4584 w4586]
      tunnel: [w4491 w4507 w4584 w4586] -> w4481
      tunnel: [_ _ TRUE _] -> w4480
      tunnel: [w4488 w4505 w4582 w4585] -> w4479
      tunnel: w4478 -> [w4493 w4519 w4582 w4585]
      tunnel: [enum16{"init", "MAIN", "Panel Close"}."MAIN" w4514 _ _] -> w4476
      frame "init" {
        n3499 = local read "C3 :"() -> (w4483:refnum<visa-resource-name>)
        n3500 = Bundle By Name(cluster=w4493, "Heave and Surge COM Port:"=w4483) -> (w4492:T18)
        n3501 = call "Instrument fgv uno.vi"("Enum"=T31."INIT", "error in (no error) 2"=w4496, "INPUT"=w4492) -> ("error"=w4494:errorcluster, "output"=w4490:T18)  [unwired: 6 in, 1 out]
        n3502 = case shown="Error" w4494 {
          selector: w4494 -> [w4498 _]
          tunnel: [w4498 w4502] -> w4491
          tunnel: w4490 -> [w4497 w4500]
          tunnel: [w4497 w4499] -> w4489
          frame No Error {
          }
          frame Error {
            n3503 = call "Instrument fgv uno.vi"("Enum"=T31."ERROR INIT", "INPUT"=w4500) -> ("error"=w4503:errorcluster, "output"=w4499:T18)  [unwired: 7 in, 1 out]
            n3504 = call <vilib>:"Clear Errors.vi"("error in (no error)"=w4503) -> ("error out"=w4502:errorcluster)  [unwired: 5 in, 1 out]
          }
        }
        n3505 = local read "LastCom Humidity"() -> (w4486:string)
        n3506 = Unbundle By Name(w4489) -> ("Heave COM Status 2"=→"COM Status":bool, "Error Heave"=→"Error":errorcluster)  [unwired: 1 out]
        n3507 = Bundle By Name(cluster=w4489, "LastCom"=w4486) -> (w4488:T18)
      }
      frame "MAIN" {
        n3508 = Unbundle By Name(w4519) -> ("Com Port 2"=w4509:refnum<visa-resource-name>)
        n3509 = local read "C3 :"() -> (w4510:refnum<visa-resource-name>)
        n3510 = local write "COM Port Humidity :"(w4509) -> ()
        n3511 = Bundle By Name(cluster=w4519, "Heave and Surge COM Port:"=w4510) -> (w4518:T18)
        n3512 = Equal?(x=w4509, y=w4510) -> (x = y?=w4523:bool)
        n3513 = case shown="True" w4523 {
          tunnel: [w4538 w4555] -> w4508
          tunnel: w4520 -> [w4539 w4561]
          tunnel: w4518 -> [w4537 w4559]
          tunnel: [w4536 w4554] -> w4506
          frame False {
            n3514 = call <vilib>:"Clear Errors.vi"("error in (no error)"=w4539) -> ("error out"=w4535:errorcluster)  [unwired: 5 in, 1 out]
            n3515 = call "Instrument fgv uno.vi"("Enum"=T31."ERROR INIT", "error in (no error) 2"=w4535, "INPUT"=w4537) -> ("error"=w4541:errorcluster, "output"=w4536:T18)  [unwired: 6 in, 1 out]
            n3516 = call <vilib>:"Clear Errors.vi"("error in (no error)"=w4541) -> ("error out"=w4538:errorcluster)  [unwired: 5 in, 1 out]
          }
          frame True {
            n3517 = call "Instrument fgv uno.vi"("Enum"=T31."READ", "error in (no error) 2"=w4561, "INPUT"=w4559) -> ("error"=w4560:errorcluster, "output"=w4553:T18)  [unwired: 6 in, 1 out]
            n3518 = Bundle By Name(cluster=w4553, "String 36"="WRITE HUMIDITY") -> (w4552:T18)
            n3519 = case shown="True" "Write Humidity" {
              selector: "Write Humidity" -> [_ w4581]
              tunnel: w4560 -> [w4574 w4580]
              tunnel: [w4574 w4579] -> w4550
              tunnel: w4552 -> [w4573 w4577]
              tunnel: [w4573 w4576] -> w4549
              frame False {
              }
              frame True {
                n3520 = Not(x=w4581) -> (.not. x?=w4575:bool)
                n3521 = local write "Write Humidity"(w4575) -> ()
                n3522 = call "Instrument fgv uno.vi"("Enum"=T31."MANUAL WRITE", "error in (no error) 2"=w4580, "INPUT"=w4577) -> ("error"=w4579:errorcluster, "output"=w4576:T18)  [unwired: 6 in, 1 out]
              }
            }
            n3523 = Array Size(array="WriteHumidity") -> (size(s)=w4547:i32)
            n3524 = Greater Than 0?(x=w4547) -> (x > 0?=w4546:bool)
            n3525 = call "Instrument fgv uno.vi"("Enum"=T31."WRITE", "error in (no error) 2"=w4550, "WriteCC1"="WriteHumidity", "INPUT"=w4549) -> ("error"=w4557:errorcluster, "WriteCC1 2"=w4548:string[], "output"=w4556:T18)  [unwired: 5 in]
            n3526 = case shown="True" w4546 {
              tunnel: w4548 -> [_ w4563]
              frame False {
              }
              frame True {
                n3527 = local write "WriteHumidity"(w4563) -> ()
              }
            }
            n3528 = case shown="No Error" w4557 {
              selector: w4557 -> [w4564 w4567]
              tunnel: w4556 -> [w4565 w4572]
              tunnel: [w4565 w4571] -> w4554
              tunnel: [w4564 w4569] -> w4555
              frame No Error {
              }
              frame Error {
                n3529 = call <vilib>:"Clear Errors.vi"("error in (no error)"=w4567) -> ("error out"=w4566:errorcluster)  [unwired: 5 in, 1 out]
                n3530 = call "Instrument fgv uno.vi"("Enum"=T31."ERROR INIT", "error in (no error) 2"=w4566, "INPUT"=w4572) -> ("error"=w4570:errorcluster, "output"=w4571:T18)  [unwired: 6 in, 1 out]
                n3531 = call <vilib>:"Clear Errors.vi"("error in (no error)"=w4570) -> ("error out"=w4569:errorcluster)  [unwired: 5 in, 1 out]
              }
            }
            n3532 = Unbundle By Name(w4554) -> ("LastCom"=→"LastCom Humidity":string, "Read Heave and Surge"=→"Read HUMIDITY":string)
          }
        }
        n3533 = Unbundle By Name(w4506) -> ("Heave COM Status 2"=w4522:bool, "Error Heave"=w4511:errorcluster, "Bytes at Heave Port"=→"Bytes at Humidity Port  2":dbl)  [unwired: 1 out]
        n3534 = Unbundle By Name(w4511) -> ("status"=→"Humidity Port":bool)
        n3535 = Not(x=w4522) -> (.not. x?=w4512:bool)
        n3536 = local write "Error"(w4511) -> ()
        n3537 = local read "Quit"() -> (w4515:bool)
        n3538 = local write "COM Status"(w4512) -> ()
        n3539 = Select(t=enum16{"init", "MAIN", "Panel Close"}."Panel Close", s=w4515, f=enum16{"init", "MAIN", "Panel Close"}."MAIN") -> (s? t:f=w4514:enum16{"init", "MAIN", "Panel Close"})
        n3540 = local read "Humidity 2"() -> (w4504:bool)
        n3541 = case shown="True" w4504 {
          selector: w4504 -> [_ w4526]
          tunnel: w4508 -> [w4524 w4531]
          tunnel: [w4524 w4530] -> w4507
          tunnel: w4506 -> [w4525 w4529]
          tunnel: [w4525 w4528] -> w4505
          frame False {
          }
          frame True {
            n3542 = Not(x=w4526) -> (.not. x?=→"Humidity 2":bool)
            n3543 = call <vilib>:"Clear Errors.vi"("error in (no error)"=w4531) -> ("error out"=w4534:errorcluster)  [unwired: 5 in, 1 out]
            n3544 = call "Instrument fgv uno.vi"("Enum"=T31."ERROR INIT", "error in (no error) 2"=w4534, "INPUT"=w4529) -> ("error"=w4532:errorcluster, "output"=w4528:T18)  [unwired: 6 in, 1 out]
            n3545 = call <vilib>:"Clear Errors.vi"("error in (no error)"=w4532) -> ("error out"=w4530:errorcluster)  [unwired: 5 in, 1 out]
          }
        }
      }
      frame "Panel Close" {
      }
      frame Default {
      }
    }
  }
  n3546 = while {
    stop <- w4588 stop-if-true
    n3547 = call <vilib>:"High Resolution Polling Wait.vi"("seconds to wait"=0.05) -> ()  [unwired: 10 in, 1 out]
    n3548 = disable-structure shown="Enabled" {
      frame Disabled {
        n3549 = local read "Read HUMIDITY"() -> (w4589:string)
        n3550 = Spreadsheet String To Array(delimiter (Tab)=",", format string="", spreadsheet string=w4589, array type (2D Dbl)=string[] []) -> (array=w4608:string[])
        n3551 = for {
          tunnel: w4608 -> [w4617] mode=indexing
          tunnel: string[] ["STATE;", "SET;", "RH;", "T;", "AMB_RH;", "AMB_T;", "PUMP;", "FAN_IN;", "FAN_OUT;", "DEHUM;", "CURRENT;", "STALL;"] -> [w4616] mode=indexing
          tunnel: [w4615] -> w4607 mode=indexing
          n3552 = Match Pattern(string=w4617, regular expression=w4616) -> (after substring=w4615:string)  [unwired: 1 in, 3 out]
        }
        n3553 = Index Array(array=w4607) -> (element #1=w4606:string, element #2=w4605:string, element #3=w4597:string, element #4=w4596:string, element #5=w4595:string, element #6=w4604:string, element #7=w4603:string, element #8=w4602:string, element #9=w4601:string, element #10=w4600:string, element #11=w4599:string, element #12=w4598:string)  [unwired: 12 in]
        n3554 = Fract/Exp String To Number(string=w4597) -> (number=w4590:dbl)  [unwired: 3 in, 1 out]
        n3555 = Fract/Exp String To Number(string=w4595) -> (number=w4594:dbl)  [unwired: 3 in, 1 out]
        n3556 = local write "Ambient Humidity :"(w4594) -> ()
        n3557 = Equal?(x=w4590, y=0.0) -> (x = y?=w4592:bool)
        n3558 = case shown="True" w4592 {
          tunnel: [w4613 w4614] -> w4591
          tunnel: w4590 -> [w4613 _]
          frame False {
            (unwired) 0.0
            "Humidity temp" <- w4613
          }
          frame True {
            n3559 = local read "Humidity temp"() -> (w4614:dbl)
          }
        }
        "RH Numeric:" <- w4591
      }
      frame Enabled {
        n3560 = local read "Read HUMIDITY"() -> (w4637:string)
        n3561 = Spreadsheet String To Array(delimiter (Tab)=",", format string="", spreadsheet string=w4637, array type (2D Dbl)=dbl[] []) -> (array=w4633:dbl[])
        n3562 = Index Array(array=w4633) -> (element #1=→"STATE :":dbl, element #2=→"SET :":dbl, element #3=w4618:dbl, element #4=→"T :":dbl, element #5=→"AMB_RH :":dbl, element #6=→"AMB_T :":dbl, element #7=→"PUMP :":dbl, element #8=→"FAN_IN :":dbl, element #9=→"FAN_OUT :":dbl, element #10=→"DEHUM :":dbl, element #11=→"CURRENT :":dbl, element #12=→"STALL":dbl)  [unwired: 12 in]
        "RH :" <- w4618
        n3563 = Equal?(x=w4618, y=0.0) -> (x = y?=w4621:bool)
        n3564 = case shown="False" w4621 {
          tunnel: [w4638 w4639] -> w4622
          tunnel: w4618 -> [w4638 _]
          frame False {
            "Humidity temp 2" <- w4638
          }
          frame True {
            n3565 = local read "Humidity temp 2"() -> (w4639:dbl)
          }
        }
        n3566 = local write "RH Numeric:"(w4622) -> ()
      }
    }
    n3567 = local read "Quit"() -> (w4588:bool)
  }
  n3568 = while {
    shift-right: [w4645] -> _
    shift-left: _ -> [w4646]
    shift-right: [w4643] -> _
    shift-left: T20 {"Read Uno"="", "Bytes at Heave Port"=0.0, "UNO COM Port:"="COM9", "UNO COM Port: 2"="COM7", "Residual Due"="", "UNO COM Status 2"=TRUE, "UNO COM Status"=TRUE, "Port 2"=TRUE, "Sway PPR"=6400.0, "Surge PPR"=6400.0, "Heave PPR"=6400.0, "Sway Pitch"=2.0, "Surge Pitch"=3.0, "Heave Pitch"=4.0, "Sway Pulses/mm"=320.0, "Surge Pulses/mm"=1600.0, "Heave Pulses/mm"=1600.0, "inner loop"=0.0, "Read Heave and Surge 2"="", "String 36"="", "Write S"=FALSE, "WriteCC1"=[""], "Heave COM Loop"=0, "LastCom"="", "EXIT"=FALSE, "Error Heave"={"status"=TRUE, "code"=-1073807343, "source"=""}} -> [w4642]
    shift-right: [w4640] -> _
    shift-left: enum16{"init", "MAIN", "Panel Close"}."init" -> [w4641]
    stop <- w4644 stop-if-true
    # "UNO CODE LOGIC"
    n3569 = case shown="\"MAIN\"" w4641 {
      tunnel: w4646 -> [w4660 w4679 w4735 w4737]
      tunnel: [w4655 w4684 w4735 w4737] -> w4645
      tunnel: [_ _ TRUE _] -> w4644
      tunnel: [w4651 w4682 w4733 w4736] -> w4643
      tunnel: w4642 -> [w4657 w4678 w4733 w4736]
      tunnel: [enum16{"init", "MAIN", "Panel Close"}."MAIN" w4673 _ _] -> w4640
      frame "init" {
        n3570 = local read "Com Port 1"() -> (w4647:refnum<visa-resource-name>)
        n3571 = Bundle By Name(cluster=w4657, "UNO COM Port:"=w4647) -> (w4656:T20)
        n3572 = call "Instrument fgv.vi"("Enum"=T31."INIT", "error in (no error) 2"=w4660, "INPUT"=w4656) -> ("error"=w4658:errorcluster, "output"=w4654:T18)  [unwired: 6 in, 1 out]
        n3573 = case shown="Error" w4658 {
          selector: w4658 -> [w4662 _]
          tunnel: [w4662 w4666] -> w4655
          tunnel: w4654 -> [w4661 w4664]
          tunnel: [w4661 w4663] -> w4652
          frame No Error {
          }
          frame Error {
            n3574 = call "Instrument fgv.vi"("Enum"=T31."ERROR INIT", "INPUT"=w4664) -> ("error"=w4667:errorcluster, "output"=w4663:T18)  [unwired: 7 in, 1 out]
            n3575 = call <vilib>:"Clear Errors.vi"("error in (no error)"=w4667) -> ("error out"=w4666:errorcluster)  [unwired: 5 in, 1 out]
          }
        }
        n3576 = local read "LastCom UNO"() -> (w4649:string)
        n3577 = Unbundle By Name(w4652) -> ("Heave COM Status 2"=→"Instrument Status":bool, "Error Heave"=→"Error  2":errorcluster)  [unwired: 1 out]
        n3578 = Bundle By Name(cluster=w4652, "LastCom"=w4649) -> (w4651:T18)
      }
      frame "MAIN" {
        n3579 = Unbundle By Name(w4678) -> ("UNO COM Port: 2"=w4668:refnum<visa-resource-name>)
        n3580 = local read "Com Port 1"() -> (w4669:refnum<visa-resource-name>)
        n3581 = local write "COM Port UNO :"(w4668) -> ()
        n3582 = Equal?(x=w4668, y=w4669) -> (x = y?=w4685:bool)
        n3583 = Bundle By Name(cluster=w4678, "UNO COM Port:"=w4669) -> (w4677:T20)
        n3584 = case shown="True" w4685 {
          tunnel: [w4689 w4706] -> w4684
          tunnel: w4679 -> [w4690 w4712]
          tunnel: w4677 -> [w4688 w4710]
          tunnel: [w4687 w4705] -> w4682
          frame False {
            n3585 = call <vilib>:"Clear Errors.vi"("error in (no error)"=w4690) -> ("error out"=w4686:errorcluster)  [unwired: 5 in, 1 out]
            n3586 = call "Instrument fgv.vi"("Enum"=T31."ERROR INIT", "error in (no error) 2"=w4686, "INPUT"=w4688) -> ("error"=w4692:errorcluster, "output"=w4687:T18)  [unwired: 6 in, 1 out]
            n3587 = call <vilib>:"Clear Errors.vi"("error in (no error)"=w4692) -> ("error out"=w4689:errorcluster)  [unwired: 5 in, 1 out]
          }
          frame True {
            n3588 = call "Instrument fgv.vi"("Enum"=T31."READ", "error in (no error) 2"=w4712, "INPUT"=w4710) -> ("error"=w4711:errorcluster, "output"=w4704:T18)  [unwired: 6 in, 1 out]
            n3589 = Bundle By Name(cluster=w4704, "String 36"="WRITE UNO") -> (w4703:T18)
            n3590 = case shown="True" "Write" {
              selector: "Write" -> [_ w4727]
              tunnel: w4711 -> [w4725 w4732]
              tunnel: [w4725 w4731] -> w4701
              tunnel: w4703 -> [w4724 w4729]
              tunnel: [w4724 w4728] -> w4700
              frame False {
              }
              frame True {
                n3591 = Not(x=w4727) -> (.not. x?=w4726:bool)
                n3592 = local write "Write"(w4726) -> ()
                n3593 = call "Instrument fgv.vi"("Enum"=T31."MANUAL WRITE", "error in (no error) 2"=w4732, "INPUT"=w4729) -> ("error"=w4731:errorcluster, "output"=w4728:T18)  [unwired: 6 in, 1 out]
              }
            }
            n3594 = Array Size(array="Write UNO") -> (size(s)=w4698:i32)
            n3595 = Greater Than 0?(x=w4698) -> (x > 0?=w4697:bool)
            n3596 = call "Instrument fgv.vi"("Enum"=T31."WRITE", "error in (no error) 2"=w4701, "WriteCC1"="Write UNO", "INPUT"=w4700) -> ("error"=w4708:errorcluster, "WriteCC1 2"=w4699:string[], "output"=w4707:T18)  [unwired: 5 in]
            n3597 = case shown="True" w4697 {
              tunnel: w4699 -> [_ w4714]
              frame False {
              }
              frame True {
                n3598 = local write "Write UNO"(w4714) -> ()
              }
            }
            n3599 = case shown="Error" w4708 {
              selector: w4708 -> [w4715 w4718]
              tunnel: w4707 -> [w4716 w4723]
              tunnel: [w4716 w4722] -> w4705
              tunnel: [w4715 w4720] -> w4706
              frame No Error {
              }
              frame Error {
                n3600 = call <vilib>:"Clear Errors.vi"("error in (no error)"=w4718) -> ("error out"=w4717:errorcluster)  [unwired: 5 in, 1 out]
                n3601 = call "Instrument fgv.vi"("Enum"=T31."ERROR INIT", "error in (no error) 2"=w4717, "INPUT"=w4723) -> ("error"=w4721:errorcluster, "output"=w4722:T18)  [unwired: 6 in, 1 out]
                n3602 = call <vilib>:"Clear Errors.vi"("error in (no error)"=w4721) -> ("error out"=w4720:errorcluster)  [unwired: 5 in, 1 out]
              }
            }
            n3603 = Unbundle By Name(w4705) -> ("LastCom"=→"LastCom UNO":string, "Read Heave and Surge"=→"Read UNO":string)
          }
        }
        n3604 = Unbundle By Name(w4682) -> ("Heave COM Status 2"=w4683:bool, "Heave COM Status"=w4672:bool, "Error Heave"=w4670:errorcluster, "Bytes at Heave Port"=→"Bytes at Humidity Port":dbl)
        n3605 = Not(x=w4672) -> (.not. x?=w4680:bool)
        n3606 = Not(x=w4683) -> (.not. x?=w4671:bool)
        n3607 = local write "Instrument Status"(w4680) -> ()
        n3608 = local write "Error  2"(w4670) -> ()
        n3609 = local write "Port 1a"(w4672) -> ()
        n3610 = local read "Quit"() -> (w4674:bool)
        n3611 = local write "COM Status"(w4671) -> ()
        n3612 = Select(t=enum16{"init", "MAIN", "Panel Close"}."Panel Close", s=w4674, f=enum16{"init", "MAIN", "Panel Close"}."MAIN") -> (s? t:f=w4673:enum16{"init", "MAIN", "Panel Close"})
      }
      frame "Panel Close" {
      }
      frame Default {
      }
    }
  }
